vi "FlexMag - 23-03-2023.vi"() -> ()   [LabVIEW 2018] (continued)
                                frame True {
                                }
                                }
                                n20789 = local read "coating start"() -> (w24946:bool)
                                n20790 = local read "abort ch3"() -> (w24940:bool)
                                n20791 = Not(x=w24946) -> (.not. x?=w24945:bool)
                                n20792 = Compound Arithmetic op=OR(w24947, w24945, w24940) -> (w24944:bool)
                                }
                                }
                                }
                                }
                                frame True {
                                }
                                }
                                }
                                frame #2 {
                                n20793 = local read "abort ch3"() -> (w24956:bool)
                                n20794 = case shown="False" w24956 {
                                frame False {
                                n20795 = local read "coating start"() -> (w24957:bool)
                                n20796 = case shown="True" w24957 {
                                frame False {
                                }
                                frame True {
                                n20797 = Wait (ms)(milliseconds to wait=u32 100) -> ()  [unwired: 1 out]
                                "coating ch3 led 5" <- TRUE ("coating ch2 led 1")
                                }
                                }
                                }
                                frame True {
                                }
                                }
                                }
                                }
                                }
                                frame #6 {
                                # "cc close"
                                n20798 = stacked-sequence {
                                frame #0 {
                                n20799 = local read "abort ch3"() -> (w24960:bool)
                                n20800 = case shown="False" w24960 {
                                frame False {
                                n20801 = local read "coating start"() -> (w24961:bool)
                                n20802 = case shown="True" w24961 {
                                frame False {
                                }
                                frame True {
                                n20803 = while {
                                i -> [w24964]
                                stop <- w24966 stop-if-true
                                n20804 = Greater Or Equal?(x=w24964, y=100) -> (x >= y?=w24965:bool)
                                n20805 = case shown="True" w24965 {
                                frame False {
                                }
                                frame True {
                                n20806 = local write "Warning Message"("Automatic Coating Process is canceled !\nCH3 ColdCathode couldn't be closed.." ("Warning Message")) -> ()
                                n20807 = local write "coating error"(TRUE ("coating error")) -> ()
                                }
                                }
                                n20808 = local read "CH3_CC_DI"() -> (w24970:bool)
                                n20809 = case shown="True" w24970 {
                                tunnel: [TRUE ("CH2_WFC_DO") FALSE ("CH2_WFC_DO")] -> w24969
                                frame False {
                                }
                                frame True {
                                n20810 = Wait Until Next ms Multiple(millisecond multiple=u32 200) -> ()  [unwired: 1 out]
                                n20811 = local write "CH3_CC_DO"(FALSE ("coating error")) -> ()
                                }
                                }
                                n20812 = local read "coating start"() -> (w24968:bool)
                                n20813 = local read "abort ch3"() -> (w24962:bool)
                                n20814 = Not(x=w24968) -> (.not. x?=w24967:bool)
                                n20815 = Compound Arithmetic op=OR(w24969, w24967, w24962) -> (w24966:bool)
                                }
                                }
                                }
                                }
                                frame True {
                                }
                                }
                                }
                                frame #1 {
                                n20816 = local read "abort ch3"() -> (w24977:bool)
                                n20817 = case shown="False" w24977 {
                                frame False {
                                n20818 = local read "coating start"() -> (w24978:bool)
                                n20819 = case shown="True" w24978 {
                                frame False {
                                }
                                frame True {
                                n20820 = Wait (ms)(milliseconds to wait=u32 100) -> ()  [unwired: 1 out]
                                "coating ch3 led 6" <- TRUE ("coating ch2 led 1")
                                }
                                }
                                }
                                frame True {
                                }
                                }
                                }
                                }
                                }
                                frame #7 {
                                # "baratron bv open"
                                n20821 = stacked-sequence {
                                frame #0 {
                                n20822 = local read "abort ch3"() -> (w24981:bool)
                                n20823 = case shown="False" w24981 {
                                frame False {
                                n20824 = local read "coating start"() -> (w24982:bool)
                                n20825 = case shown="True" w24982 {
                                frame False {
                                }
                                frame True {
                                n20826 = while {
                                i -> [w24985]
                                stop <- w24987 stop-if-true
                                n20827 = Greater Or Equal?(x=w24985, y=100) -> (x >= y?=w24986:bool)
                                n20828 = case shown="True" w24986 {
                                frame False {
                                }
                                frame True {
                                n20829 = local write "Warning Message"("Automatic Coating Process is canceled !\nCH3 Baratron Gauge Block Valve couldn't be opned.." ("Warning Message")) -> ()
                                n20830 = local write "coating error"(TRUE ("coating error")) -> ()
                                }
                                }
                                n20831 = local read "CH3_BG_BV_DI"() -> (w24991:bool)
                                n20832 = case shown="False" w24991 {
                                tunnel: [FALSE ("CH2_WFC_DO") TRUE ("CH2_WFC_DO")] -> w24990
                                frame False {
                                n20833 = Wait Until Next ms Multiple(millisecond multiple=u32 200) -> ()  [unwired: 1 out]
                                n20834 = local write "CH3_BG_BV_DO"(TRUE ("coating error")) -> ()
                                }
                                frame True {
                                }
                                }
                                n20835 = local read "coating start"() -> (w24989:bool)
                                n20836 = local read "abort ch3"() -> (w24983:bool)
                                n20837 = Not(x=w24989) -> (.not. x?=w24988:bool)
                                n20838 = Compound Arithmetic op=OR(w24990, w24988, w24983) -> (w24987:bool)
                                }
                                }
                                }
                                }
                                frame True {
                                }
                                }
                                }
                                frame #1 {
                                n20839 = local read "abort ch3"() -> (w24998:bool)
                                n20840 = case shown="False" w24998 {
                                frame False {
                                n20841 = local read "coating start"() -> (w24999:bool)
                                n20842 = case shown="True" w24999 {
                                frame False {
                                }
                                frame True {
                                n20843 = Wait (ms)(milliseconds to wait=u32 100) -> ()  [unwired: 1 out]
                                "coating ch3 led 7" <- TRUE ("coating ch2 led 1")
                                }
                                }
                                }
                                frame True {
                                }
                                }
                                }
                                }
                                }
                                frame #8 {
                                # "ar sov open"
                                n20844 = stacked-sequence {
                                frame #0 {
                                n20845 = local read "abort ch3"() -> (w25002:bool)
                                n20846 = case shown="False" w25002 {
                                frame False {
                                n20847 = local read "coating start"() -> (w25003:bool)
                                n20848 = case shown="True" w25003 {
                                frame False {
                                }
                                frame True {
                                n20849 = while {
                                i -> [w25006]
                                stop <- w25008 stop-if-true
                                n20850 = Greater Or Equal?(x=w25006, y=100) -> (x >= y?=w25007:bool)
                                n20851 = case shown="True" w25007 {
                                frame False {
                                }
                                frame True {
                                n20852 = local write "Warning Message"("Automatic Coating Process is canceled !\nCH3 SoV Ar couldn't be opened.." ("Warning Message")) -> ()
                                n20853 = local write "coating error"(TRUE ("coating error")) -> ()
                                }
                                }
                                n20854 = local read "CH3_SoV_Ar_DI"() -> (w25012:bool)
                                n20855 = case shown="False" w25012 {
                                tunnel: [FALSE ("CH2_WFC_DO") TRUE ("CH2_WFC_DO")] -> w25011
                                frame False {
                                n20856 = Wait Until Next ms Multiple(millisecond multiple=u32 200) -> ()  [unwired: 1 out]
                                n20857 = local write "CH3_SoV_Ar_DO"(TRUE ("coating error")) -> ()
                                }
                                frame True {
                                }
                                }
                                n20858 = local read "coating start"() -> (w25010:bool)
                                n20859 = local read "abort ch3"() -> (w25004:bool)
                                n20860 = Not(x=w25010) -> (.not. x?=w25009:bool)
                                n20861 = Compound Arithmetic op=OR(w25011, w25009, w25004) -> (w25008:bool)
                                }
                                }
                                }
                                }
                                frame True {
                                }
                                }
                                }
                                frame #1 {
                                n20862 = local read "abort ch3"() -> (w25019:bool)
                                n20863 = case shown="False" w25019 {
                                frame False {
                                n20864 = local read "coating start"() -> (w25020:bool)
                                n20865 = case shown="True" w25020 {
                                frame False {
                                }
                                frame True {
                                n20866 = Wait (ms)(milliseconds to wait=u32 100) -> ()  [unwired: 1 out]
                                "coating ch3 led 8" <- TRUE ("coating ch2 led 1")
                                }
                                }
                                }
                                frame True {
                                }
                                }
                                }
                                }
                                }
                                frame #9 {
                                # "mfc set"
                                n20867 = stacked-sequence {
                                frame #0 {
                                n20868 = local read "abort ch3"() -> (w25023:bool)
                                n20869 = case shown="False" w25023 {
                                frame False {
                                n20870 = local read "coating start"() -> (w25024:bool)
                                n20871 = case shown="True" w25024 {
                                frame False {
                                }
                                frame True {
                                n20872 = flat-sequence {
                                frame #0 {
                                n20873 = local read "R Ar set sccm"() -> (w25026:dbl)
                                n20874 = local write "ch3 argon mfc set"(w25026) -> ()
                                n20875 = Wait (ms)(milliseconds to wait=u32 300) -> ()  [unwired: 1 out]
                                }
                                frame #1 {
                                n20876 = local write "ch3 ar set auto"(TRUE ("ch2 ar set auto")) -> ()
                                }
                                }
                                }
                                }
                                }
                                frame True {
                                }
                                }
                                }
                                frame #1 {
                                n20877 = local read "abort ch3"() -> (w25028:bool)
                                n20878 = case shown="False" w25028 {
                                frame False {
                                n20879 = local read "coating start"() -> (w25029:bool)
                                n20880 = case shown="True" w25029 {
                                frame False {
                                }
                                frame True {
                                n20881 = while {
                                i -> [w25039]
                                stop <- w25041 stop-if-true
                                n20882 = local read "R Ar set sccm"() -> (w25035:dbl)
                                n20883 = Greater Or Equal?(x=w25039, y=50) -> (x >= y?=w25040:bool)
                                n20884 = case shown="True" w25040 {
                                frame False {
                                }
                                frame True {
                                n20885 = local write "Warning Message"("Automatic Coating Process is canceled !\nCH3  MFC Ar flow problem..." ("Warning Message")) -> ()
                                n20886 = local write "coating error"(TRUE ("coating error")) -> ()
                                }
                                }
                                n20887 = local read "ch3 argon mfc actual"() -> (w25036:dbl)
                                n20888 = Add(x=w25035, y=5.0) -> (x+y=w25032:dbl)
                                n20889 = Subtract(x=w25035, y=5.0) -> (x-y=w25031:dbl)
                                n20890 = In Range and Coerce(upper limit=w25032, x=w25036, lower limit=w25031) -> (In Range?=w25030:bool)  [unwired: 1 out]
                                n20891 = case shown="False" w25030 {
                                tunnel: [FALSE ("CH2_WFC_DO") TRUE ("CH2_WFC_DO")] -> w25044
                                frame False {
                                n20892 = Wait Until Next ms Multiple(millisecond multiple=u32 1000) -> ()  [unwired: 1 out]
                                n20893 = local write "ch3 ar set auto"(TRUE ("coating error")) -> ()
                                }
                                frame True {
                                }
                                }
                                n20894 = local read "coating start"() -> (w25043:bool)
                                n20895 = local read "abort ch3"() -> (w25037:bool)
                                n20896 = Not(x=w25043) -> (.not. x?=w25042:bool)
                                n20897 = Compound Arithmetic op=OR(w25044, w25042, w25037) -> (w25041:bool)
                                }
                                }
                                }
                                }
                                frame True {
                                }
                                }
                                }
                                frame #2 {
                                n20898 = local read "abort ch3"() -> (w25051:bool)
                                n20899 = case shown="False" w25051 {
                                frame False {
                                n20900 = local read "coating start"() -> (w25052:bool)
                                n20901 = case shown="True" w25052 {
                                frame False {
                                }
                                frame True {
                                n20902 = Wait (ms)(milliseconds to wait=u32 100) -> ()  [unwired: 1 out]
                                "coating ch3 led 9" <- TRUE ("coating ch2 led 1")
                                }
                                }
                                }
                                frame True {
                                }
                                }
                                }
                                }
                                }
                                frame #10 {
                                # "baratron pressure set"
                                n20903 = stacked-sequence {
                                frame #0 {
                                n20904 = local read "abort ch3"() -> (w25055:bool)
                                n20905 = case shown="False" w25055 {
                                frame False {
                                n20906 = local read "coating start"() -> (w25056:bool)
                                n20907 = case shown="True" w25056 {
                                frame False {
                                }
                                frame True {
                                n20908 = flat-sequence {
                                frame #0 {
                                n20909 = local read "R Pressure set mbar"() -> (w25057:dbl)
                                n20910 = Wait (ms)(milliseconds to wait=u32 300) -> ()  [unwired: 1 out]
                                n20911 = local write "pcgv3 set pressure value mbar"(w25057) -> ()
                                }
                                frame #1 {
                                n20912 = local write "pcgv3 auto set pressure"(TRUE ("ch2 ar set auto")) -> ()
                                }
                                }
                                }
                                }
                                }
                                frame True {
                                }
                                }
                                }
                                frame #1 {
                                n20913 = local read "abort ch3"() -> (w25060:bool)
                                n20914 = case shown="False" w25060 {
                                frame False {
                                n20915 = local read "coating start"() -> (w25061:bool)
                                n20916 = case shown="True" w25061 {
                                frame False {
                                }
                                frame True {
                                n20917 = while {
                                i -> [w25071]
                                stop <- w25073 stop-if-true
                                n20918 = local read "R Pressure set mbar"() -> (w25067:dbl)
                                n20919 = Greater Or Equal?(x=w25071, y=50) -> (x >= y?=w25072:bool)
                                n20920 = case shown="True" w25072 {
                                frame False {
                                }
                                frame True {
                                n20921 = local write "Warning Message"("Automatic Coating Process is canceled !\nCH3 Baratron Pressure Set problem..." ("Warning Message")) -> ()
                                n20922 = local write "coating error"(TRUE ("coating error")) -> ()
                                }
                                }
                                n20923 = local read "Ch3_baratron_pressure_mbar"() -> (w25068:dbl)
                                n20924 = Add(x=w25067, y=0.003) -> (x+y=w25064:dbl)
                                n20925 = Subtract(x=w25067, y=0.003) -> (x-y=w25063:dbl)
                                n20926 = In Range and Coerce(upper limit=w25064, x=w25068, lower limit=w25063) -> (In Range?=w25062:bool)  [unwired: 1 out]
                                n20927 = case shown="False" w25062 {
                                tunnel: [FALSE ("CH2_WFC_DO") TRUE ("CH2_WFC_DO")] -> w25076
                                frame False {
                                n20928 = Wait Until Next ms Multiple(millisecond multiple=u32 1000) -> ()  [unwired: 1 out]
                                n20929 = local write "pcgv3 auto set pressure"(TRUE ("coating error")) -> ()
                                }
                                frame True {
                                }
                                }
                                n20930 = local read "coating start"() -> (w25075:bool)
                                n20931 = local read "abort ch3"() -> (w25069:bool)
                                n20932 = Not(x=w25075) -> (.not. x?=w25074:bool)
                                n20933 = Compound Arithmetic op=OR(w25076, w25074, w25069) -> (w25073:bool)
                                }
                                }
                                }
                                }
                                frame True {
                                }
                                }
                                }
                                frame #2 {
                                n20934 = local read "abort ch3"() -> (w25083:bool)
                                n20935 = case shown="False" w25083 {
                                frame False {
                                n20936 = local read "coating start"() -> (w25084:bool)
                                n20937 = case shown="True" w25084 {
                                frame False {
                                }
                                frame True {
                                n20938 = Wait (ms)(milliseconds to wait=u32 100) -> ()  [unwired: 1 out]
                                "coating ch3 led 10" <- TRUE ("coating ch2 led 1")
                                }
                                }
                                }
                                frame True {
                                }
                                }
                                }
                                }
                                }
                                frame #11 {
                                # "power set"
                                n20939 = stacked-sequence {
                                frame #0 {
                                n20940 = local read "abort ch3"() -> (w25087:bool)
                                n20941 = case shown="False" w25087 {
                                frame False {
                                n20942 = local read "coating start"() -> (w25088:bool)
                                n20943 = case shown="True" w25088 {
                                frame False {
                                }
                                frame True {
                                n20944 = flat-sequence {
                                frame #0 {
                                n20945 = local write "Dc_auto_off"(TRUE ("Dc_auto_off")) -> ()
                                }
                                frame #1 {
                                n20946 = local write "Set DC Power auto"(200.0 ("Set DC Power")) -> ()
                                n20947 = Wait (ms)(milliseconds to wait=u32 2000) -> ()  [unwired: 1 out]
                                }
                                frame #2 {
                                n20948 = local write "Dc_auto_set"(TRUE ("Dc_auto_set")) -> ()
                                }
                                }
                                }
                                }
                                }
                                frame True {
                                }
                                }
                                }
                                frame #1 {
                                n20949 = local read "abort ch3"() -> (w25093:bool)
                                n20950 = case shown="False" w25093 {
                                frame False {
                                n20951 = local read "coating start"() -> (w25094:bool)
                                n20952 = case shown="True" w25094 {
                                frame False {
                                }
                                frame True {
                                n20953 = flat-sequence {
                                frame #0 {
                                n20954 = local read "R dc step length 20"() -> (w25108:dbl)
                                n20955 = local read "R web thickness"() -> (w25121:dbl)
                                n20956 = local read "R dc step length 11"() -> (w25099:dbl)
                                n20957 = local read "R dc step length 12"() -> (w25100:dbl)
                                n20958 = local read "R dc step length 13"() -> (w25101:dbl)
                                n20959 = local read "R dc step length 14"() -> (w25102:dbl)
                                n20960 = local read "R dc step length 15"() -> (w25103:dbl)
                                n20961 = local read "R dc step length 16"() -> (w25104:dbl)
                                n20962 = local read "R dc step length 17"() -> (w25105:dbl)
                                n20963 = local read "R dc step length 18"() -> (w25106:dbl)
                                n20964 = local read "R dc step length 19"() -> (w25107:dbl)
                                n20965 = local read "R core diameter"() -> (w25122:dbl)
                                n20966 = local read "R dc step length 10"() -> (w25110:dbl)
                                n20967 = local read "R tension value"() -> (w25120:dbl)
                                n20968 = local read "R dc step length 1"() -> (w25119:dbl)
                                n20969 = local read "R dc step length 2"() -> (w25118:dbl)
                                n20970 = local read "R dc step length 3"() -> (w25117:dbl)
                                n20971 = local read "R dc step length 4"() -> (w25116:dbl)
                                n20972 = local read "R dc step length 5"() -> (w25115:dbl)
                                n20973 = local read "R dc step length 6"() -> (w25114:dbl)
                                n20974 = local read "R dc step length 7"() -> (w25113:dbl)
                                n20975 = local read "R dc step length 8"() -> (w25112:dbl)
                                n20976 = local read "R dc step length 9"() -> (w25111:dbl)
                                n20977 = local read "R web speed"() -> (w25095:dbl)
                                n20978 = local write "web speed"(w25095) -> ()
                                n20979 = local write "initial right diameter"(w25122) -> ()
                                n20980 = local write "web thickness"(w25121) -> ()
                                n20981 = local write "tension value"(w25120) -> ()
                                n20982 = local write "setpoint"(w25095) -> ()
                                n20983 = Compound Arithmetic op=ADD(w25099, w25100, w25101, w25102, w25103, w25104, w25105, w25106, w25107, w25108) -> (w25097:dbl)
                                n20984 = Compound Arithmetic op=ADD(w25119, w25118, w25117, w25116, w25115, w25114, w25113, w25112, w25111, w25110) -> (w25098:dbl)
                                n20985 = Compound Arithmetic op=ADD(w25098, w25097) -> (w25096:dbl)
                                n20986 = local write "target interval"(w25096) -> ()
                                n20987 = Wait (ms)(milliseconds to wait=u32 500) -> ()  [unwired: 1 out]
                                }
                                frame #1 {
                                n20988 = Wait (ms)(milliseconds to wait=u32 500) -> ()  [unwired: 1 out]
                                }
                                frame #2 {
                                n20989 = local write "calculate"(TRUE ("calculate")) -> ()
                                }
                                }
                                }
                                }
                                }
                                frame True {
                                }
                                }
                                }
                                frame #2 {
                                n20990 = local read "abort ch3"() -> (w25125:bool)
                                n20991 = case shown="False" w25125 {
                                frame False {
                                n20992 = local read "coating start"() -> (w25126:bool)
                                n20993 = case shown="True" w25126 {
                                frame False {
                                }
                                frame True {
                                n20994 = flat-sequence {
                                frame #0 {
                                n20995 = while {
                                i -> [w25131]
                                stop <- w25127 stop-if-true
                                n20996 = local read "coating start"() -> (w25135:bool)
                                n20997 = local read "calculate"() -> (w25136:bool)
                                n20998 = local read "abort ch3"() -> (w25134:bool)
                                n20999 = Greater Or Equal?(x=w25131, y=60) -> (x >= y?=w25128:bool)
                                n21000 = Not(x=w25136) -> (.not. x?=w25132:bool)
                                n21001 = Not(x=w25135) -> (.not. x?=w25133:bool)
                                n21002 = Wait Until Next ms Multiple(millisecond multiple=u32 1000) -> ()  [unwired: 1 out]
                                n21003 = Compound Arithmetic op=OR(w25128, w25132, w25133, w25134) -> (w25127:bool)
                                }
                                }
                                frame #1 {
                                n21004 = local read "R DC number steps"() -> (w25137:dbl)
                                n21005 = Wait (ms)(milliseconds to wait=u32 1000) -> ()  [unwired: 1 out]
                                n21006 = local write "step count"(w25137) -> ()
                                }
                                }
                                }
                                }
                                }
                                frame True {
                                }
                                }
                                }
                                frame #3 {
                                n21007 = local read "abort ch3"() -> (w25139:bool)
                                n21008 = case shown="False" w25139 {
                                frame False {
                                n21009 = local read "coating start"() -> (w25140:bool)
                                n21010 = case shown="True" w25140 {
                                frame False {
                                }
                                frame True {
                                n21011 = flat-sequence {
                                frame #0 {
                                n21012 = local read "dep. for?"() -> (w25141:bool)
                                n21013 = case shown="False" w25141 {
                                frame False {
                                n21014 = local write "back roll"(TRUE ("back roll")) -> ()
                                }
                                frame True {
                                n21015 = local write "forward roll"(TRUE ("forward roll")) -> ()
                                }
                                }
                                }
                                frame #1 {
                                n21016 = Wait (ms)(milliseconds to wait=u32 1000) -> ()  [unwired: 1 out]
                                }
                                frame #2 {
                                n21017 = while {
                                i -> [w25150]
                                stop <- w25147 stop-if-true
                                n21018 = local read "CH3_Motor DO"() -> (w25146:bool)
                                n21019 = local read "coating start"() -> (w25153:bool)
                                n21020 = Wait Until Next ms Multiple(millisecond multiple=u32 1000) -> ()  [unwired: 1 out]
                                n21021 = local read "abort ch3"() -> (w25152:bool)
                                n21022 = Greater Or Equal?(x=w25150, y=60) -> (x >= y?=w25145:bool)
                                n21023 = Not(x=w25153) -> (.not. x?=w25151:bool)
                                n21024 = local write "Dc_auto_on"(w25146) -> ()
                                n21025 = local write "stop coating"(w25145) -> ()
                                n21026 = Compound Arithmetic op=OR(w25146, w25151, w25152, w25145) -> (w25147:bool)
                                }
                                }
                                frame #3 {
                                n21027 = Wait (ms)(milliseconds to wait=u32 1000) -> ()  [unwired: 1 out]
                                }
                                }
                                }
                                }
                                }
                                frame True {
                                }
                                }
                                }
                                frame #4 {
                                n21028 = local read "abort ch3"() -> (w25155:bool)
                                n21029 = case shown="False" w25155 {
                                frame False {
                                n21030 = local read "coating start"() -> (w25156:bool)
                                n21031 = case shown="True" w25156 {
                                frame False {
                                }
                                frame True {
                                }
                                }
                                }
                                frame True {
                                }
                                }
                                }
                                frame #5 {
                                n21032 = local read "abort ch3"() -> (w25157:bool)
                                n21033 = case shown="False" w25157 {
                                frame False {
                                n21034 = local read "coating start"() -> (w25158:bool)
                                n21035 = case shown="True" w25158 {
                                frame False {
                                }
                                frame True {
                                n21036 = Wait (ms)(milliseconds to wait=u32 100) -> ()  [unwired: 1 out]
                                "coating ch3 led 11" <- TRUE ("coating ch2 led 1")
                                }
                                }
                                }
                                frame True {
                                }
                                }
                                }
                                }
                                }
                                frame #12 {
                                # "power steps"
                                n21037 = disable-structure shown="Enabled" {
                                frame Disabled {
                                n21038 = stacked-sequence {
                                frame #0 {
                                n21039 = local read "abort ch3"() -> (w25161:bool)
                                n21040 = case shown="False" w25161 {
                                frame False {
                                n21041 = local read "coating start"() -> (w25162:bool)
                                n21042 = case shown="True" w25162 {
                                frame False {
                                }
                                frame True {
                                n21043 = local read "R dc step length 1"() -> (w25165:dbl)
                                n21044 = Greater?(x=w25165, y=0.0) -> (0:w25164:bool)
                                n21045 = case shown="True" w25164 {
                                frame False {
                                }
                                frame True {
                                n21046 = flat-sequence {
                                frame #0 {
                                n21047 = local read "R dc step length 1"() -> (w25172:dbl)
                                n21048 = local read "R dc step power 1"() -> (w25167:dbl)
                                n21049 = local read "R web speed"() -> (w25171:dbl)
                                n21050 = Divide(x=w25172, y=w25171) -> (x/y=w25170:dbl)
                                n21051 = local write "Set DC Power ch2"(w25167) -> ()
                                n21052 = Multiply(x=w25170, y=60) -> (x*y=w25168:dbl)
                                n21053 = Wait (ms)(milliseconds to wait=u32 100) -> ()  [unwired: 1 out]
                                n21054 = local write "time counting"(w25168) -> ()
                                }
                                frame #1 {
                                n21055 = local write "Dc_auto_set"(TRUE ("Dc_auto_set")) -> ()
                                }
                                frame #2 {
                                n21056 = while {
                                stop <- w25175 stop-if-true
                                n21057 = local read "time counting"() -> (w25181:dbl)
                                n21058 = Wait Until Next ms Multiple(millisecond multiple=u32 1000) -> ()  [unwired: 1 out]
                                n21059 = local read "coating start"() -> (w25179:bool)
                                n21060 = local read "abort ch3"() -> (w25177:bool)
                                n21061 = Decrement(x=w25181) -> (x-1=w25180:dbl)
                                n21062 = local write "time counting"(w25180) -> ()
                                n21063 = Not(x=w25179) -> (.not. x?=w25178:bool)
                                n21064 = Less Or Equal To 0?(x=w25180) -> (x <= 0?=w25176:bool)
                                n21065 = Compound Arithmetic op=OR(w25176, w25178, w25177) -> (w25175:bool)
                                }
                                }
                                }
                                }
                                }
                                }
                                }
                                }
                                frame True {
                                }
                                }
                                }
                                frame #1 {
                                n21066 = local read "abort ch3"() -> (w25182:bool)
                                n21067 = case shown="False" w25182 {
                                frame False {
                                n21068 = local read "coating start"() -> (w25183:bool)
                                n21069 = case shown="True" w25183 {
                                frame False {
                                }
                                frame True {
                                n21070 = local read "R dc step length 2"() -> (w25186:dbl)
                                n21071 = Greater?(x=w25186, y=0.0) -> (0:w25185:bool)
                                n21072 = case shown="True" w25185 {
                                frame False {
                                }
                                frame True {
                                n21073 = flat-sequence {
                                frame #0 {
                                n21074 = local read "R dc step length 2"() -> (w25193:dbl)
                                n21075 = local read "R dc step power 2"() -> (w25188:dbl)
                                n21076 = local read "R web speed"() -> (w25192:dbl)
                                n21077 = Divide(x=w25193, y=w25192) -> (x/y=w25191:dbl)
                                n21078 = local write "Set DC Power ch2"(w25188) -> ()
                                n21079 = Multiply(x=w25191, y=60) -> (x*y=w25189:dbl)
                                n21080 = Wait (ms)(milliseconds to wait=u32 100) -> ()  [unwired: 1 out]
                                n21081 = local write "time counting"(w25189) -> ()
                                }
                                frame #1 {
                                n21082 = local write "Dc_auto_set"(TRUE ("Dc_auto_set")) -> ()
                                }
                                frame #2 {
                                n21083 = while {
                                stop <- w25196 stop-if-true
                                n21084 = local read "time counting"() -> (w25202:dbl)
                                n21085 = local read "coating start"() -> (w25200:bool)
                                n21086 = local read "abort ch3"() -> (w25198:bool)
                                n21087 = Wait Until Next ms Multiple(millisecond multiple=u32 1000) -> ()  [unwired: 1 out]
                                n21088 = Decrement(x=w25202) -> (x-1=w25201:dbl)
                                n21089 = local write "time counting"(w25201) -> ()
                                n21090 = Not(x=w25200) -> (.not. x?=w25199:bool)
                                n21091 = Less Or Equal To 0?(x=w25201) -> (x <= 0?=w25197:bool)
                                n21092 = Compound Arithmetic op=OR(w25197, w25199, w25198) -> (w25196:bool)
                                }
                                }
                                }
                                }
                                }
                                }
                                }
                                }
                                frame True {
                                }
                                }
                                }
                                frame #2 {
                                n21093 = local read "abort ch3"() -> (w25203:bool)
                                n21094 = case shown="False" w25203 {
                                frame False {
                                n21095 = local read "coating start"() -> (w25204:bool)
                                n21096 = case shown="True" w25204 {
                                frame False {
                                }
                                frame True {
                                n21097 = local read "R dc step length 3"() -> (w25207:dbl)
                                n21098 = Greater?(x=w25207, y=0.0) -> (0:w25206:bool)
                                n21099 = case shown="True" w25206 {
                                frame False {
                                }
                                frame True {
                                n21100 = flat-sequence {
                                frame #0 {
                                n21101 = local read "R dc step length 3"() -> (w25214:dbl)
                                n21102 = local read "R dc step power 3"() -> (w25209:dbl)
                                n21103 = local read "R web speed"() -> (w25213:dbl)
                                n21104 = Divide(x=w25214, y=w25213) -> (x/y=w25212:dbl)
                                n21105 = local write "Set DC Power ch2"(w25209) -> ()
                                n21106 = Multiply(x=w25212, y=60) -> (x*y=w25210:dbl)
                                n21107 = Wait (ms)(milliseconds to wait=u32 100) -> ()  [unwired: 1 out]
                                n21108 = local write "time counting"(w25210) -> ()
                                }
                                frame #1 {
                                n21109 = local write "Dc_auto_set"(TRUE ("Dc_auto_set")) -> ()
                                }
                                frame #2 {
                                n21110 = while {
                                stop <- w25217 stop-if-true
                                n21111 = local read "time counting"() -> (w25223:dbl)
                                n21112 = local read "coating start"() -> (w25221:bool)
                                n21113 = Wait Until Next ms Multiple(millisecond multiple=u32 1000) -> ()  [unwired: 1 out]
                                n21114 = local read "abort ch3"() -> (w25219:bool)
                                n21115 = Decrement(x=w25223) -> (x-1=w25222:dbl)
                                n21116 = local write "time counting"(w25222) -> ()
                                n21117 = Not(x=w25221) -> (.not. x?=w25220:bool)
                                n21118 = Less Or Equal To 0?(x=w25222) -> (x <= 0?=w25218:bool)
                                n21119 = Compound Arithmetic op=OR(w25218, w25220, w25219) -> (w25217:bool)
                                }
                                }
                                }
                                }
                                }
                                }
                                }
                                }
                                frame True {
                                }
                                }
                                }
                                frame #3 {
                                n21120 = local read "abort ch3"() -> (w25224:bool)
                                n21121 = case shown="False" w25224 {
                                frame False {
                                n21122 = local read "coating start"() -> (w25225:bool)
                                n21123 = case shown="True" w25225 {
                                frame False {
                                }
                                frame True {
                                n21124 = local read "R dc step length 4"() -> (w25228:dbl)
                                n21125 = Greater?(x=w25228, y=0.0) -> (0:w25227:bool)
                                n21126 = case shown="True" w25227 {
                                frame False {
                                }
                                frame True {
                                n21127 = flat-sequence {
                                frame #0 {
                                n21128 = local read "R dc step length 4"() -> (w25235:dbl)
                                n21129 = local read "R dc step power 4"() -> (w25230:dbl)
                                n21130 = local read "R web speed"() -> (w25234:dbl)
                                n21131 = Divide(x=w25235, y=w25234) -> (x/y=w25233:dbl)
                                n21132 = local write "Set DC Power ch2"(w25230) -> ()
                                n21133 = Wait (ms)(milliseconds to wait=u32 100) -> ()  [unwired: 1 out]
                                n21134 = Multiply(x=w25233, y=60) -> (x*y=w25231:dbl)
                                n21135 = local write "time counting"(w25231) -> ()
                                }
                                frame #1 {
                                n21136 = local write "Dc_auto_set"(TRUE ("Dc_auto_set")) -> ()
                                }
                                frame #2 {
                                n21137 = while {
                                stop <- w25238 stop-if-true
                                n21138 = local read "time counting"() -> (w25244:dbl)
                                n21139 = local read "coating start"() -> (w25242:bool)
                                n21140 = local read "abort ch3"() -> (w25240:bool)
                                n21141 = Wait Until Next ms Multiple(millisecond multiple=u32 1000) -> ()  [unwired: 1 out]
                                n21142 = Decrement(x=w25244) -> (x-1=w25243:dbl)
                                n21143 = local write "time counting"(w25243) -> ()
                                n21144 = Not(x=w25242) -> (.not. x?=w25241:bool)
                                n21145 = Less Or Equal To 0?(x=w25243) -> (x <= 0?=w25239:bool)
                                n21146 = Compound Arithmetic op=OR(w25239, w25241, w25240) -> (w25238:bool)
                                }
                                }
                                }
                                }
                                }
                                }
                                }
                                }
                                frame True {
                                }
                                }
                                }
                                frame #4 {
                                n21147 = local read "abort ch3"() -> (w25245:bool)
                                n21148 = case shown="False" w25245 {
                                frame False {
                                n21149 = local read "coating start"() -> (w25246:bool)
                                n21150 = case shown="True" w25246 {
                                frame False {
                                }
                                frame True {
                                n21151 = local read "R dc step length 5"() -> (w25249:dbl)
                                n21152 = Greater?(x=w25249, y=0.0) -> (0:w25248:bool)
                                n21153 = case shown="True" w25248 {
                                frame False {
                                }
                                frame True {
                                n21154 = flat-sequence {
                                frame #0 {
                                n21155 = local read "R dc step length 5"() -> (w25256:dbl)
                                n21156 = local read "R dc step power 5"() -> (w25251:dbl)
                                n21157 = local read "R web speed"() -> (w25255:dbl)
                                n21158 = Divide(x=w25256, y=w25255) -> (x/y=w25254:dbl)
                                n21159 = Wait (ms)(milliseconds to wait=u32 100) -> ()  [unwired: 1 out]
                                n21160 = local write "Set DC Power ch2"(w25251) -> ()
                                n21161 = Multiply(x=w25254, y=60) -> (x*y=w25252:dbl)
                                n21162 = local write "time counting"(w25252) -> ()
                                }
                                frame #1 {
                                n21163 = local write "Dc_auto_set"(TRUE ("Dc_auto_set")) -> ()
                                }
                                frame #2 {
                                n21164 = while {
                                stop <- w25259 stop-if-true
                                n21165 = local read "time counting"() -> (w25265:dbl)
                                n21166 = local read "coating start"() -> (w25263:bool)
                                n21167 = Wait Until Next ms Multiple(millisecond multiple=u32 1000) -> ()  [unwired: 1 out]
                                n21168 = local read "abort ch3"() -> (w25261:bool)
                                n21169 = Decrement(x=w25265) -> (x-1=w25264:dbl)
                                n21170 = local write "time counting"(w25264) -> ()
                                n21171 = Not(x=w25263) -> (.not. x?=w25262:bool)
                                n21172 = Less Or Equal To 0?(x=w25264) -> (x <= 0?=w25260:bool)
                                n21173 = Compound Arithmetic op=OR(w25260, w25262, w25261) -> (w25259:bool)
                                }
                                }
                                }
                                }
                                }
                                }
                                }
                                }
                                frame True {
                                }
                                }
                                }
                                frame #5 {
                                n21174 = local read "abort ch3"() -> (w25266:bool)
                                n21175 = case shown="False" w25266 {
                                frame False {
                                n21176 = local read "coating start"() -> (w25267:bool)
                                n21177 = case shown="True" w25267 {
                                frame False {
                                }
                                frame True {
                                n21178 = local read "R dc step length 6"() -> (w25270:dbl)
                                n21179 = Greater?(x=w25270, y=0.0) -> (0:w25269:bool)
                                n21180 = case shown="True" w25269 {
                                frame False {
                                }
                                frame True {
                                n21181 = flat-sequence {
                                frame #0 {
                                n21182 = local read "R dc step length 6"() -> (w25277:dbl)
                                n21183 = local read "R dc step power 6"() -> (w25272:dbl)
                                n21184 = local read "R web speed"() -> (w25276:dbl)
                                n21185 = Wait (ms)(milliseconds to wait=u32 100) -> ()  [unwired: 1 out]
                                n21186 = Divide(x=w25277, y=w25276) -> (x/y=w25275:dbl)
                                n21187 = local write "Set DC Power ch2"(w25272) -> ()
                                n21188 = Multiply(x=w25275, y=60) -> (x*y=w25273:dbl)
                                n21189 = local write "time counting"(w25273) -> ()
                                }
                                frame #1 {
                                n21190 = local write "Dc_auto_set"(TRUE ("Dc_auto_set")) -> ()
                                }
                                frame #2 {
                                n21191 = while {
                                stop <- w25280 stop-if-true
                                n21192 = local read "time counting"() -> (w25286:dbl)
                                n21193 = local read "coating start"() -> (w25284:bool)
                                n21194 = local read "abort ch3"() -> (w25282:bool)
                                n21195 = Wait Until Next ms Multiple(millisecond multiple=u32 1000) -> ()  [unwired: 1 out]
                                n21196 = Decrement(x=w25286) -> (x-1=w25285:dbl)
                                n21197 = local write "time counting"(w25285) -> ()
                                n21198 = Not(x=w25284) -> (.not. x?=w25283:bool)
                                n21199 = Less Or Equal To 0?(x=w25285) -> (x <= 0?=w25281:bool)
                                n21200 = Compound Arithmetic op=OR(w25281, w25283, w25282) -> (w25280:bool)